vi "UHR-Fleezers Control (host) - 12.7.vi"() -> ()   [LabVIEW 2012] (continued)
              shift-left: _ -> [w2929]
              n2002 = case shown="True" w2938 {
                selector: w2938 -> [w2945 _]
                tunnel: w2940 -> [_ w2954]
                tunnel: w2939 -> [_ w2952]
                tunnel: [w2945 w2950] -> w2937
                tunnel: [w2944 w2949] -> w2936
                tunnel: [w2943 w2948] -> w2935
                tunnel: [w2942 w2947] -> w2934
                tunnel: [w2941 w2946] -> w2933
                tunnel: w2932 -> [w2944 _]
                tunnel: w2931 -> [w2943 _]
                tunnel: w2930 -> [w2942 _]
                tunnel: w2929 -> [w2941 _]
                frame False {
                }
                frame True {
                  n2003 = Unbundle(w2954) -> (w2953:T33)
                  n2004 = call "isclickinwindow.vi"("Image Param"=w2953, "Point32"=w2952) -> ("4 Y"=w2946:i32, "3 Height"=w2947:i32, "2 X"=w2948:i32, "1 Width"=w2949:i32, "In image?"=w2951:bool)  [unwired: 1 in]
                  n2005 = Not(x=w2951) -> (.not. x?=w2950:bool)
                }
              }
            }
            n2006 = Not(x=w2904) -> (.not. x?=w2903:bool)
            n2007 = case shown="True" w2903 {
              tunnel: w2901 -> [_ w2968]
              tunnel: w2899 -> [_ w2967]
              tunnel: w2902 -> [_ w2966]
              tunnel: w2900 -> [_ w2965]
              frame False {
              }
              frame True {
                w2955 = FALSE ("Get Point")
                n2008 = local read "Scan lines (y)"() -> (w2970:u64)
                n2009 = disable-structure shown="Disabled" {
                  frame Disabled {
                  }
                  frame Enabled {
                  }
                }
                n2010 = local read "Actual MCL Inc (V)"() -> (w2964:dbl)
                n2011 = local read "Scan steps (MCL)"() -> (w2969:u64)
                n2012 = Divide "Y Pix/step"(x=w2965, y=w2970) -> (x/y=w2977:dbl)
                n2013 = Divide "Y V/pix"(x=w2964, y=w2977) -> (x/y=w2976:dbl)
                n2014 = Divide "Y half step offset"(x=w2964, y=2.0) -> (x/y=w2978:dbl)
                n2015 = Divide "X pix/step"(x=w2966, y=w2969) -> (x/y=w2975:dbl)
                n2016 = Negate(x=w2978) -> (-x=w2979:dbl)
                n2017 = local read "Initial Y"() -> (w2985:dbl)
                n2018 = Multiply(x=w2967, y=w2976) -> (x*y=w2986:dbl)
                n2019 = Divide "X half step offset"(x=w2964, y=2.0) -> (x/y=w2972:dbl)
                n2020 = Divide "X V/pix"(x=w2964, y=w2975) -> (x/y=w2974:dbl)
                n2021 = Multiply(x=w2964, y=w2969) -> (x*y=w2981:dbl)
                n2022 = Compound Arithmetic op=ADD(w2979, w2986, w2985) -> (w2956:dbl)
                "Pointer Y (V)" <- w2956
                n2023 = Multiply(x=w2974, y=w2968) -> (x*y=w2983:dbl)
                n2024 = Negate(x=w2972) -> (-x=w2971:dbl)
                n2025 = local read "Initial X"() -> (w2984:dbl)
                n2026 = Negate(x=w2983) -> (-x=w2982:dbl)
                n2027 = Compound Arithmetic op=ADD(w2971, w2981, w2984, w2982) -> (w2957:dbl)
                "Pointer X (V)" <- w2957
                n2028 = case shown="True" "Set High F Confocal Spot (X-Y)" {
                  tunnel: w2957 -> [_ w2987]
                  tunnel: w2956 -> [_ w2988]
                  frame False {
                  }
                  frame True {
                    "Confocal Y 2 (V)" <- w2988
                    "Confocal X 2 (V)" <- w2987
                  }
                }
                n2029 = Or(x="Set X Only", y="Set Confocal Spot (X-Y)") -> (x .or. y?=w2960:bool)
                n2030 = Or(x="Set Confocal Spot (X-Y)", y="Set Y Only") -> (x .or. y?=w2959:bool)
                n2031 = case shown="True" w2960 {
                  tunnel: w2957 -> [_ w2989]
                  frame False {
                  }
                  frame True {
                    n2032 = property on="AO2" class="Slide (strict)"("Val(Sgnl)"=w2989) -> ()  [unwired: 2 in, 2 out]
                    "Confocal X 1 (V)" <- w2989
                  }
                }
                n2033 = case shown="True" w2959 {
                  tunnel: w2956 -> [_ w2990]
                  frame False {
                  }
                  frame True {
                    n2034 = property on="AO1" class="Slide (strict)"("Val(Sgnl)"=w2990) -> ()  [unwired: 2 in, 2 out]
                    "Confocal Y 1 (V)" <- w2990
                  }
                }
                n2035 = local write "Set High F Confocal Spot (X-Y)"(w2955) -> ()
                n2036 = local write "Set Confocal Spot (X-Y)"(w2955) -> ()
                n2037 = local write "Set X Only"(w2955) -> ()
                n2038 = local write "Set Y Only"(w2955) -> ()
              }
            }
          }
          frame 3 {
            n2039 = local read "BD 2 Frequency 1 (MHz)"() -> (w2991:dbl)
            n2040 = local read "BD 1 Frequency 1 (MHz)"() -> (w2992:dbl)
            n2041 = local write "Manipulating Trap"(TRUE ("Manipulating Trap")) -> ()
            n2042 = local write "Coords"(T7 {"Horizontal"=0, "Vertical"=0} ("Coords")) -> ()
            n2043 = while {
              tunnel: w2997 -> [w3002]
              tunnel: w2995 -> [w3001]
              tunnel: w2993 -> [w3000]
              tunnel: w2992 -> [w2999]
              tunnel: w2991 -> [w2998]
              stop <- w3003 stop-if-true
              n2044 = event shown="[0] \"Pane\": Mouse Move" {
                selector: _ -> [_ _]
                dyn-events: _ -> [_ _]
                timeout: _ -> [_ _]
                tunnel: ["Force Manip Abort" w3067] -> w3003
                tunnel: w3002 -> [w3010 _]
                tunnel: w3001 -> [w3008 _]
                tunnel: w3000 -> [w3007 _]
                tunnel: w2999 -> [w3006 _]
                tunnel: w2998 -> [w3005 _]
                event Mouse Move {
                  n2045 = event-data() -> ("Time"=w3011:u32, "Coords"=w3012:T7)  [unwired: 3 out]
                  n2046 = Less?(x=w3011, y=w3010) -> (x < y?=w3009:bool)
                  n2047 = case "Makes sure old motion events prior to mouse click aren't used" shown="False" w3009 {
                    tunnel: w3012 -> [w3054 _]
                    tunnel: w3008 -> [w3055 _]
                    tunnel: w3007 -> [w3032 _]
                    tunnel: w3006 -> [w3028 _]
                    tunnel: w3005 -> [w3027 _]
                    frame False {
                      n2048 = Subtract(x=w3054, y=w3055) -> (x-y=w3053:T7)
                      "Coords" <- w3053
                      n2049 = local read "Y RF Frequency Limits (MHz)"() -> (w3013:T16)
                      n2050 = To Double Precision Float(number=w3053) -> (double precision float=w3052:cluster{"Horizontal":dbl, "Vertical":dbl})
                      n2051 = Multiply(x=cluster{"Horizontal":dbl, "Vertical":dbl} {"Horizontal"=-1.0, "Vertical"=1.0}, y="Manipulation Scaling") -> (x*y=w3048:cluster{"Horizontal":dbl, "Vertical":dbl})
                      n2052 = local read "X RF Frequency Limits (MHz)"() -> (w3014:T16)
                      n2053 = Multiply(x=w3052, y=w3048) -> (x*y=w3050:cluster{"Horizontal":dbl, "Vertical":dbl})
                      n2054 = Unbundle By Name(w3050) -> ("Horizontal"=w3045:dbl, "Vertical"=w3049:dbl)
                      n2055 = Unbundle By Name(w3013) -> ("Maximum"=w3016:dbl, "Minimum"=w3015:dbl)
                      n2056 = Boolean To (0,1)(Boolean="Manip. X?") -> (0, 1=w3043:i16)
                      n2057 = Boolean To (0,1)(Boolean="Manip. Y?") -> (0, 1=w3040:i16)
                      n2058 = local read "BD 1 Frequency 2 (MHz)"() -> (w3030:dbl)
                      n2059 = Multiply(x=w3049, y=w3040) -> (x*y=w3042:dbl)
                      n2060 = Multiply(x=w3043, y=w3045) -> (x*y=w3046:dbl)
                      n2061 = local read "BD 2 Frequency 2 (MHz)"() -> (w3029:dbl)
                      n2062 = Unbundle By Name(w3014) -> ("Maximum"=w3018:dbl, "Minimum"=w3017:dbl)
                      n2063 = Add(x=w3027, y=w3042) -> (x+y=w3020:dbl)
                      n2064 = Add(x=w3028, y=w3046) -> (x+y=w3022:dbl)
                      n2065 = In Range and Coerce(upper limit=w3018, x=w3022, lower limit=w3017) -> (coerced(x)=w3021:dbl)  [unwired: 1 out]
                      n2066 = In Range and Coerce(upper limit=w3016, x=w3020, lower limit=w3015) -> (coerced(x)=w3019:dbl)  [unwired: 1 out]
                      n2067 = Subtract(x=w3021, y=w3030) -> (x-y=w3039:dbl)
                      n2068 = Subtract(x=w3019, y=w3029) -> (x-y=w3038:dbl)
                      n2069 = Square(x=w3039) -> (x^2=w3037:dbl)
                      n2070 = Square(x=w3038) -> (x^2=w3036:dbl)
                      n2071 = Add(x=w3037, y=w3036) -> (x+y=w3035:dbl)
                      n2072 = Square Root(x=w3035) -> (sqrt(x)=w3031:dbl)
                      n2073 = In Range and Coerce(upper limit="Limit Max (MHz)", x=w3031, lower limit="Limit Min (MHz)") -> (In Range?=w3024:bool)  [unwired: 1 out]
                      n2074 = Not(x="Limits Enable") -> (.not. x?=w3023:bool)
                      n2075 = Or(x=w3024, y=w3023) -> (x .or. y?=w3025:bool)
                      n2076 = case shown="True" w3025 {
                        tunnel: w3032 -> [_ w3065]
                        tunnel: w3031 -> [_ w3056]
                        tunnel: w3021 -> [_ w3063]
                        tunnel: w3030 -> [_ w3062]
                        tunnel: w3019 -> [_ w3061]
                        tunnel: w3029 -> [_ w3060]
                        tunnel: w3014 -> [_ w3058]
                        tunnel: w3013 -> [_ w3057]
                        frame False {
                        }
                        frame True {
                          n2077 = local read "BD 1 Frequency 3 (MHz)"() -> (w3064:dbl)
                          n2078 = local read "BD 2 Frequency 3 (MHz)"() -> (w3059:dbl)
                          n2079 = local write "Trap Delta (MHz)"(w3056) -> ()
                          n2080 = call "set RF board frequency - interlace.vi"("Board 2 Frequency Limits"=w3057, "Board 1 Frequency Limits"=w3058, "FPGA VI Reference In"=w3065, "Board 2 Frequency 3 (MHz)"=w3059, "Board 1 Frequency 3 (MHz)"=w3064, "Board 2 Frequency 2 (MHz)"=w3060, "Board 2 Frequency 1 (MHz)"=w3061, "Board 1 Frequency 2 (MHz)"=w3062, "Board 1 Frequency 1  (MHz)"=w3063) -> ()  [unwired: 1 in, 2 out]
                          n2081 = local write "BD 2 Frequency 1 (MHz)"(w3061) -> ()
                          n2082 = local write "BD 1 Frequency 1 (MHz)"(w3063) -> ()
                        }
                      }
                    }
                    frame True {
                    }
                  }
                }
                event Mouse Up {
                  n2083 = event-data() -> ("Button"=w3066:u16)  [unwired: 8 out]
                  n2084 = case shown="3" w3066 {
                    tunnel: [FALSE TRUE] -> w3067
                    frame 0, Default {
                    }
                    frame 3 {
                      n2085 = local read "Trap Delta (MHz)"() -> (w3069:dbl)
                      n2086 = property on="Initial delta (MHz)" class="DigNum (strict)"("Val(Sgnl)"=w3069) -> ()  [unwired: 2 in, 2 out]
                      n2087 = local write "Manipulating Trap"(FALSE ("Manipulating Trap")) -> ()
                    }
                  }
                }
              }
            }
          }
        }
      }
      event Mouse Move {
        n2088 = event-data() -> ()  [unwired: 6 out]
      }
    }
    n2089 = local read "Stop All"() -> (w2885:bool)
    n2090 = node-c288() -> ()  [unwired: 2 out]
  }
  n2091 = timed-loop "Main data acquisition loop (get data, process data for display, and save data to disk)" {
    tunnel: w17 -> [w3381]
    tunnel: w89 -> [w3380]
    tunnel: [w3410] -> w293
    tunnel: [w3405] -> w291
    timing: w201 -> [_]
    timing-out: [_] -> w200
    tunnel: w106 -> [w3234]
    stop <- "Stop All" stop-if-true
    w3151 = "Initialize"
    # "Fluorescence data into FIFO for external control vi's\n(e.g., fluorescence triggering) - Duncan Nall"
    n2092 = node-c288() -> ()  [unwired: 2 out]
    n2093 = First Call?() -> (First Call?: T/F=w3186:bool)
    n2094 = Or(x="Reset", y=w3186) -> (x .or. y?=w3187:bool)
    n2095 = local read "Flushing P1"() -> (w3106:bool)
    n2096 = case "Reset data stream (manual reset or at begining of some rastering and imaging)" shown="True" w3187 {
      tunnel: w3381 -> [w4451 w4459]
      tunnel: w3380 -> [w4450 w4458]
      tunnel: [w4451 w4453] -> w3376
      tunnel: [w4450 w4452] -> w3375
      frame False {
      }
      frame True {
        w4456 = TRUE ("AI to FIFO")
        n2097 = local write "Overflow (data lost)"(FALSE ("Overflow (data lost)")) -> ()
        n2098 = call "reset FPGA DMA.vi"("error in"=w4458, "FPGA VI Reference In"=w4459) -> ("error out"=w4454:errorcluster, "FPGA VI Reference Out"=w4455:T20)
        n2099 = xnode "Read/Write Control"("FPGA VI Reference In"=w4455, "error in"=w4454, "AI to FIFO"=w4456, "APD to FIFO"=w4456) -> ("FPGA VI Reference Out"=w4453:T20, "error out"=w4452:errorcluster)
      }
    }
    n2100 = case shown="True" w3106 {
      frame False {
      }
      frame True {
        n2101 = local read "Flush rate (uL/m) P1"() -> (w3440:dbl)
        n2102 = local read "HP1 Flush Time (s)"() -> (w3449:dbl)
        n2103 = local read "DMA Update Period (s)"() -> (w3443:dbl)
        n2104 = Divide(x=w3440, y=60.0) -> (x/y=w3441:dbl)
        n2105 = Divide(x=w3449, y=w3443) -> (x/y=w3438:dbl)
        n2106 = feedback #1(0) -> (w3447:i32)
        n2107 = Increment(x=w3447) -> (x+1=w3437:i32)
        n2108 = Greater?(x=w3437, y=w3438) -> (0:w3446:bool)
        n2109 = Compound Arithmetic op=MULTIPLY(w3443, w3437, w3441) -> (→"P1 Flush Volume (uL)":dbl)
        n2110 = Divide(x=w3437, y=w3438) -> (x/y=→"P1 Flushing Bar":dbl)
        n2111 = case shown="True" w3446 {
          tunnel: w3437 -> [w3450 _]
          tunnel: [w3450 0] -> w3445
          frame False {
          }
          frame True {
            w3451 = FALSE ("Flushing P1")
            n2112 = local write "Inject Pump 1"(w3451) -> ()
            n2113 = local write "Flushing P1"(w3451) -> ()
            n2114 = property on="Clear Volume P1" class="Bool (strict)"("Val(Sgnl)"=TRUE ("Value (Signaling)")) -> ()  [unwired: 2 in, 2 out]
          }
        }
        n2115 = feedback-in #1(w3445) -> ()
      }
    }
    n2116 = Or(x="Start AOD Scan", y="Trap Raster Scan") -> (x .or. y?=w3332:bool)
    n2117 = case "Start AOM raster scan" shown="True" w3332 {
      tunnel: w3376 -> [w4301 w4311]
      tunnel: w3375 -> [w4300 w4310]
      tunnel: [w4301 w4304] -> w3374
      tunnel: [w4300 w4303] -> w3373
      frame False {
      }
      frame True {
        n2118 = case shown="True" "Restart DMA? (AOD)" {
          tunnel: [w4349 w4351] -> w4305
          tunnel: [w4348 w4350] -> w4306
          tunnel: w4311 -> [w4349 w4353]
          tunnel: w4310 -> [w4348 w4352]
          frame False {
          }
          frame True {
            n2119 = local write "Overflow (data lost)"(FALSE ("Overflow (data lost)")) -> ()
            n2120 = call "reset FPGA DMA.vi"("error in"=w4352, "FPGA VI Reference In"=w4353) -> ("error out"=w4350:errorcluster, "FPGA VI Reference Out"=w4351:T20)
          }
        }
        n2121 = local write "Trap Raster Scan"(FALSE ("Trap Raster Scan")) -> ()
        n2122 = case shown="True" "Move MCL Also?" {
          tunnel: w4306 -> [w4314 w4343]
          tunnel: w4305 -> [w4315 w4344]
          tunnel: [w4313 w4347] -> w4304
          tunnel: [w4312 w4346] -> w4303
          frame False {
            w4316 = TRUE ("AI to FIFO")
            n2123 = xnode "Read/Write Control"("FPGA VI Reference In"=w4315, "error in"=w4314, "AI to FIFO"=w4316, "APD to FIFO"=w4316, "Start scan"=w4316) -> ("FPGA VI Reference Out"=w4313:T20, "error out"=w4312:errorcluster)
          }
          frame True {
            w4340 = FALSE ("1D or 2D Scan?")
            w4345 = TRUE ("AI to FIFO")
            # "Count for MCL loop"
            # "N total cycles"
            # "N steps"
            # "V_int"
            n2124 = local read "Scan Range (nm)"() -> (w4322:dbl)
            n2125 = local read "Number of F/B Scans (AOD)"() -> (w4339:u16)
            n2126 = Sign(1:w4322) -> (0:w4321:dbl)
            n2127 = Compound Arithmetic op=MULTIPLY(w4322, "MCL Step Position Ratio", "MCL/AOM Scale Tweak") -> (w4326:dbl)
            n2128 = Negate(x=w4321) -> (-x=w4318:dbl)
            n2129 = Multiply(x=w4318, y="MCL Step Increment (V_int)") -> (x*y=w4320:dbl)
            n2130 = Divide(x=w4326, y="MCL X Cal (nm/V)") -> (x/y=w4332:dbl)
            n2131 = Multiply(x=32767.0 ("y"), y=w4332) -> (x*y=w4338:dbl)
            n2132 = local read "Total Counts (ticks)"() -> (w4323:u16)
            n2133 = local read "Cycles/step (AOD)"() -> (w4334:u64)
            n2134 = local read "Scan steps (AOD)"() -> (w4335:u64)
            n2135 = Divide(x=w4338, y=10.0) -> (x/y=w4331:dbl)
            n2136 = Divide(x=w4331, y="MCL Step Increment (V_int)") -> (x/y=w4329:dbl)
            n2137 = Absolute Value(x=w4329) -> (abs(x)=w4317:dbl)
            n2138 = Compound Arithmetic op=MULTIPLY(w4335, w4334, w4323) -> (w4330:u64)
            n2139 = local write "wait to reset values"(w4345) -> ()
            n2140 = local write "MCL Scanning"(w4345) -> ()
            n2141 = Divide(x=w4330, y=w4317) -> (x/y=w4327:dbl)
            "MCL Count" <- w4327
            n2142 = xnode "Read/Write Control"("FPGA VI Reference In"=w4344, "error in"=w4343, "Scan steps (MCL)"=w4317, "Number of scans (MCL)"=w4339, "Cycles per step (MCL)"=u64 1, "Scan freq.  increment (MCL)"=w4320, "1D or 2D Scan?"=w4340, "MCL Scan Axis"=w4340, "Cont. Scan (MCL)"=w4340, "MCL count"=w4327) -> ("FPGA VI Reference Out"=w4342:T20, "error out"=w4341:errorcluster)
            n2143 = xnode "Read/Write Control"("FPGA VI Reference In"=w4342, "error in"=w4341, "AI to FIFO"=w4345, "APD to FIFO"=w4345, "Start scan"=w4345, "Start scan (MCL)"=w4345) -> ("FPGA VI Reference Out"=w4347:T20, "error out"=w4346:errorcluster)
          }
        }
        "Raster Scanning..." <- TRUE ("Scanning...")
      }
    }
    n2144 = local read "Flushing P3"() -> (w3107:bool)
    n2145 = case "Keep track of when Harvard Pump 3 is done flushing" shown="True" w3107 {
      frame False {
      }
      frame True {
        n2146 = local read "Flush rate (uL/m) P3"() -> (w3457:dbl)
        n2147 = local read "DMA Update Period (s)"() -> (w3459:dbl)
        n2148 = local read "HP3 Flush Time (s)"() -> (w3466:dbl)
        n2149 = Divide(x=w3457, y=60.0) -> (x/y=w3455:dbl)
        n2150 = feedback #2(0) -> (w3464:i32)
        n2151 = Increment(x=w3464) -> (x+1=w3458:i32)
        n2152 = Divide(x=w3466, y=w3459) -> (x/y=w3460:dbl)
        n2153 = Greater?(x=w3458, y=w3460) -> (0:w3463:bool)
        n2154 = Compound Arithmetic op=MULTIPLY(w3459, w3458, w3455) -> (→"P3 Flush Volume (uL)":dbl)
        n2155 = case shown="True" w3463 {
          tunnel: w3458 -> [w3467 _]
          tunnel: [w3467 0] -> w3462
          frame False {
          }
          frame True {
            w3468 = FALSE ("Flushing P3")
            n2156 = local write "Inject Pump 3"(w3468) -> ()
            n2157 = local write "Flushing P3"(w3468) -> ()
            n2158 = property on="Clear Volume P3" class="Bool (strict)"("Val(Sgnl)"=TRUE ("Value (Signaling)")) -> ()  [unwired: 2 in, 2 out]
          }
        }
        n2159 = feedback-in #2(w3462) -> ()
        n2160 = Divide(x=w3458, y=w3460) -> (x/y=→"P3 Flushing Bar":dbl)
      }
    }
    n2161 = And(x="Save scans", y=w3332) -> (x .and. y?=w3372:bool)
    n2162 = Compound Arithmetic op=OR("Start MCL Scan", "Confocal Image", "Confocal Linescan") -> (w3330:bool)
    n2163 = And(x="Save Data (MCL)", y=w3330) -> (x .and. y?=w3371:bool)
    n2164 = case "Start MCL raster scan" shown="True" w3330 {
      tunnel: w3374 -> [w3913 w3929]
      tunnel: w3373 -> [w3912 w3928]
      tunnel: [w3913 w3924] -> w3233
      tunnel: [w3912 w3923] -> w3232
      tunnel: [FALSE w3922] -> w3357
      tunnel: "Start MCL Scan" -> [_ w3917]
      tunnel: "Confocal Image" -> [_ w3916]
      tunnel: "Confocal Linescan" -> [_ _]
      frame False {
      }
      frame True {
        w3922 = TRUE
        n2165 = case shown="True" "Restart DMA? (MCL)" {
          tunnel: [w3974 w3976] -> w3927
          tunnel: [w3973 w3975] -> w3926
          tunnel: w3929 -> [w3974 w3979]
          tunnel: w3928 -> [w3973 w3978]
          frame False {
          }
          frame True {
            n2166 = call "reset FPGA DMA.vi"("error in"=w3978, "FPGA VI Reference In"=w3979) -> ("error out"=w3975:errorcluster, "FPGA VI Reference Out"=w3976:T20)
            n2167 = local write "Overflow (data lost)"(FALSE ("Overflow (data lost)")) -> ()
          }
        }
        n2168 = case shown="False" w3917 {
          selector: w3917 -> [_ w3933]
          tunnel: w3916 -> [w3932 _]
          tunnel: [w3932 w3933] -> w3915
          frame False {
            n2169 = property on="2D or 1D Scan" class="Bool (strict)"("Val(Sgnl)"=w3932) -> ()  [unwired: 2 in, 2 out]
            n2170 = property on="Confocal Image" class="Bool (strict)"("Value"=FALSE ("Start Confocal Map")) -> ()  [unwired: 2 in, 2 out]
          }
          frame True {
          }
        }
        n2171 = local write "MCL Scanning"(w3922) -> ()
        n2172 = local read "AO1"() -> (w3919:dbl)
        n2173 = local read "AO2"() -> (w3918:dbl)
        n2174 = case shown="True" "Center Scan" {
          tunnel: w3927 -> [w3940 w3972]
          tunnel: w3926 -> [w3939 w3971]
          tunnel: [w3938 w3970] -> w3924
          tunnel: [w3937 w3969] -> w3923
          tunnel: [w3935 w3956] -> w3921
          tunnel: [w3934 w3955] -> w3920
          tunnel: w3919 -> [w3935 w3961]
          tunnel: w3918 -> [w3934 w3964]
          tunnel: w3915 -> [_ _]
          frame False {
            w3936 = TRUE ("AI to FIFO")
            n2175 = xnode "Read/Write Control"("FPGA VI Reference In"=w3940, "error in"=w3939, "AI to FIFO"=w3936, "APD to FIFO"=w3936, "Start scan (MCL)"=w3936) -> ("FPGA VI Reference Out"=w3938:T20, "error out"=w3937:errorcluster)
          }
          frame True {
            w3968 = TRUE ("AI to FIFO")
            n2176 = local read "Scan steps (MCL)"() -> (w3947:u64)
            n2177 = local read "Scan lines (y)"() -> (w3943:u64)
            n2178 = local read "Fast Scan Dir"() -> (w3954:bool)
            n2179 = local read "Actual MCL Inc (V)"() -> (w3944:dbl)
            n2180 = Decrement(x=w3943) -> (x-1=w3942:u64)
            n2181 = Decrement(x=w3947) -> (x-1=w3946:u64)
            n2182 = Multiply(x=w3944, y=w3942) -> (x*y=w3941:dbl)
            n2183 = Divide(x=w3941, y=2.0) -> (x/y=w3951:dbl)
            n2184 = Multiply(x=w3944, y=w3946) -> (x*y=w3945:dbl)
            n2185 = Divide(x=w3945, y=2.0) -> (x/y=w3950:dbl)
            n2186 = Select(t=w3950, s=w3954, f=w3951) -> (s? t:f=w3949:dbl)
            n2187 = Select(t=w3951, s=w3954, f=w3950) -> (s? t:f=w3953:dbl)
            n2188 = Subtract(x=w3961, y=w3953) -> (x-y=w3952:dbl)
            n2189 = Subtract(x=w3964, y=w3949) -> (x-y=w3948:dbl)
            n2190 = local read "2D or 1D Scan"() -> (w3966:bool)
            n2191 = Not(x=w3954) -> (.not. x?=w3960:bool)
            n2192 = Not(x=w3966) -> (.not. x?=w3962:bool)
            n2193 = And(x=w3954, y=w3962) -> (x .and. y?=w3963:bool)
            n2194 = And(x=w3962, y=w3960) -> (x .and. y?=w3965:bool)
            n2195 = Select(t=w3964, s=w3965, f=w3948) -> (s? t:f=w3955:dbl)
            n2196 = Select(t=w3961, s=w3963, f=w3952) -> (s? t:f=w3956:dbl)
            n2197 = call "Volt to I16.vi"("Voltage In"=w3956) -> ("I16 Voltage Out"=w3959:i16)
            n2198 = call "Volt to I16.vi"("Voltage In"=w3955) -> ("I16 Voltage Out"=w3958:i16)
            n2199 = xnode "Read/Write Control"("FPGA VI Reference In"=w3972, "error in"=w3971, "AI to FIFO"=w3968, "APD to FIFO"=w3968, "Start scan (MCL)"=w3968, "AO1"=w3959, "AO2"=w3958) -> ("FPGA VI Reference Out"=w3970:T20, "error out"=w3969:errorcluster)
          }
        }
        "Initial Y" <- w3921
        "Initial X" <- w3920
        n2200 = local write "Tab Control 6"(T3."Imaging" ("Tab Control 6")) -> ()
        "wait to reset values" <- w3922
      }
    }
    n2201 = local read "APD Elements/DMA read"() -> (w3074:u32)
    n2202 = local read "Trap AI Elements/DMA read"() -> (w3295:u32)
    n2203 = xnode "Get APD Data"("FPGA VI Reference In"=w3233, "error in"=w3232, "Number of Elements"=w3074, "Timeout (ms)"=-1) -> ("Data"=w3264:u32[], "Elements Remaining"=→"APD FIFO Elements Remaining":u32)  [unwired: 2 out]
    n2204 = local read "Trap Pos Elements/DMA read"() -> (w3229:u32)
    n2205 = xnode "Invoke Method"("FPGA VI Reference In"=w3233, "error in"=w3232, "Number of Elements"=w3229, "Timeout (ms)"=-1) -> ("Data"=w3193:u16[], "Elements Remaining"=→"Trap Pos FIFO El Remaining":u32)  [unwired: 2 out]
    n2206 = xnode "Get Trap Data"("FPGA VI Reference In"=w3233, "error in"=w3232, "Number of Elements"=w3295, "Timeout (ms)"=-1 ("Timeout")) -> ("FPGA VI Reference Out"=w3128:T20, "error out"=w3127:errorcluster, "Data"=w3194:i16[], "Elements Remaining"=w3418:u32)
    "FIFO El. Rem." <- w3418
    n2207 = local read "DMA Update Period (s)"() -> (w3296:dbl)
    n2208 = local read "Trap AI FIFO Depth"() -> (w3420:u32)
    n2209 = local read "Number of APDs"() -> (w3096:u8)
    n2210 = Decimate 1D Array(w3193) -> (w3190:u16[], w3192:u16[], w3191:u16[])
    n2211 = feedback #3(0.0) -> (w3222:dbl)
    n2212 = Add(x=w3296, y=w3222) -> (x+y=w3394:dbl)
    n2213 = feedback-in #3(w3394) -> ()
    n2214 = To Time Stamp(1:w3222) -> (0:w3221:timestamp)
    n2215 = Subtract(x=w3420, y=w3295) -> (x-y=w3419:u32)
    n2216 = To Unsigned Long Integer(number=w3190) -> (unsigned 32bit integer=w3189:u32[])
    n2217 = Join Numbers(hi=w3192, lo=w3191) -> ((hi.lo)=w3188:u32[])
    n2218 = Divide(x=w3418, y=w3419) -> (x/y=w3417:dbl)
    "Buffer Status" <- w3417
    n2219 = case "Deinterlace APD signals" shown="3, Default" w3096 {
      tunnel: [w3430 w3436] -> w3073
      tunnel: w3264 -> [w3431 w3435]
      tunnel: [w3429 w3434] -> w3072
      tunnel: [w3428 w3432] -> w3079
      frame 3, Default {
        n2220 = Decimate 1D Array "APD signals"(w3431) -> (w3430:u32[], w3429:u32[], w3428:u32[])
      }
      frame 2 {
        n2221 = Decimate 1D Array "APD signals"(w3435) -> (w3436:u32[], w3434:u32[])
        n2222 = Multiply(x=w3434, y=u32 0) -> (x*y=w3432:u32[])
      }
    }
    n2223 = Join Numbers(hi=w3189, lo=w3188) -> ((hi.lo)=w3182:u64[])
    n2224 = call "IR AOM word to freq - vec.vi"("Frequency Word In (double vec)"=w3182) -> ("Frequency Out"=w3228:dbl[])
    n2225 = Equal?(x=w3417, y=1.0) -> (x = y?=w3415:bool)
    n2226 = case "Alert buffer overflow" shown="True" w3415 {
      frame False {
      }
      frame True {
        n2227 = call <vilib>:"Beep.vi"() -> ()  [unwired: 3 in, 9 out]
        "Overflow (data lost)" <- TRUE ("Overflow (data lost)")
      }
    }
    n2228 = Decimate 1D Array(w3228) -> (w3227:dbl[], w3226:dbl[])
    n2229 = Build Array(w3227, w3226) -> (w3225:dbl[][])
    n2230 = Bundle(w3073, w3072, w3079) -> (w3077:cluster{u32[], u32[], u32[]})  [unwired: 1 in]
    n2231 = Build Array(w3073, w3072, w3079) -> (w3354:u32[][])
    n2232 = for {
      tunnel: w3073 -> [w3426] mode=indexing
      n2233 = call "Smart Buffer (DBL) 1.vi"("new element [write]"=w3426, "mode"=T21."write") -> ()  [unwired: 4 in, 6 out]
    }
    n2234 = local read "APD Integration Time (s)"() -> (w3089:dbl)
    n2235 = To Double Precision Float(number=w3354) -> (double precision float=w3355:dbl[][])
    n2236 = feedback #4 "APD3"(w3079) -> (w3095:u32[])
    n2237 = feedback #5 "APD2"(w3072) -> (w3251:u32[])
    n2238 = feedback #6 "APD1"(w3073) -> (w3353:u32[])
    n2239 = Build Array (concatenate)(w3251, w3072) -> (w3250:u32[])
    n2240 = Build Array (concatenate)(w3095, w3079) -> (w3094:u32[])
    n2241 = Build Array (concatenate)(w3353, w3073) -> (w3350:u32[])
    n2242 = for {
      tunnel: w3072 -> [w3425] mode=indexing
      n2243 = call "Smart Buffer (DBL) 2.vi"("new element [write]"=w3425, "mode"=T21."write") -> ()  [unwired: 4 in, 6 out]
    }
    n2244 = Array Size(array=w3350) -> (size(s)=w3347:i32)
    n2245 = Array Size(array=w3073) -> (size(s)=w3349:i32)
    n2246 = Multiply(x=w3349, y="APD Ave N") -> (x*y=w3348:dbl)
    n2247 = Greater?(x=w3347, y=w3348) -> (0:w3351:bool)
    n2248 = Bundle("APD 1", "APD 2", "APD 3") -> (w3387:cluster{string, string, string})  [unwired: 1 out]
    n2249 = local read "Trap Sets"() -> (w3294:u32)
    n2250 = case shown="True" w3351 {
      tunnel: w3350 -> [w3728 w3737]
      tunnel: [w3728 w3735] -> w3301
      tunnel: w3348 -> [_ w3730]
      tunnel: w3347 -> [_ w3736]
      tunnel: w3250 -> [w3727 w3734]
      tunnel: [w3727 w3733] -> w3248
      tunnel: w3094 -> [w3726 w3732]
      tunnel: [w3726 w3729] -> w3090
      frame False {
      }
      frame True {
        n2251 = Subtract(x=w3736, y=w3730) -> (x-y=w3731:dbl)
        n2252 = Array Subset "APD3"(array=w3732, index=w3731, length=w3730) -> (w3729:u32[])
        n2253 = Array Subset "APD2"(array=w3734, index=w3731, length=w3730) -> (w3733:u32[])
        n2254 = Array Subset "APD1"(array=w3737, index=w3731, length=w3730) -> (w3735:u32[])
      }
    }
    n2255 = feedback-in #4(w3090) -> ()
    n2256 = feedback-in #5(w3248) -> ()
    n2257 = feedback-in #6(w3301) -> ()
    n2258 = Cluster To Array(cluster=w3387) -> (array=w3384:string[])
    n2259 = for "APD" {
      tunnel: w3355 -> [w3984] mode=indexing
      tunnel: w3089 -> [w3991]
      tunnel: [w3987] -> w3252 mode=indexing
      tunnel: "APD Disp. Scale" -> [w3988]
      tunnel: w3384 -> [w3986] mode=indexing
      tunnel: "APD Disp. Downsample" -> [w3982]
      tunnel: [w3985] -> w3383
      workers-P: _ -> [_]
      tunnel: w3221 -> [w3981]
      n2260 = call "integrate 1D array interval - double.vi"("Ave N"=w3982, "Array In"=w3984) -> ("Array Out"=w3983:dbl[])  [unwired: 1 out]
      n2261 = Multiply(x=w3991, y=w3982) -> (x*y=w3985:dbl)
      n2262 = Divide(x=w3983, y=w3988) -> (x/y=w3989:dbl[])
      n2263 = Bundle By Name("t0"=w3981, "Y"=w3989, "dt"=w3985) -> (w3990:waveform(dbl))  [unwired: 1 out]
      n2264 = Set Waveform Attribute(5:w3986, 6:"NI_ChannelName" ("name"), 7:w3990) -> (3:w3987:waveform(dbl))  [unwired: 1 in, 2 out]
    }
    "APD Display Period (s)" <- w3383
    n2265 = Reciprocal(x=w3383) -> (1/x=→"APD Display Freq. (Hz)":dbl)
    n2266 = case "Deinterlace trap data, average down PSD" shown="2" w3294 {
      tunnel: w3194 -> [w4009 w4074]
      tunnel: [w4006 w4071] -> w3287
      tunnel: [w4009 w4073] -> w3185
      tunnel: "Detector Type" -> [w4008 w4069]
      tunnel: [w4007 w4072] -> w3286
      tunnel: [w4005 w4070] -> w3392
      frame 1, Default {
        n2267 = Divide(x=w4009, y=3276.7) -> (x/y=w4010:dbl[])
        n2268 = Decimate 1D Array(w4010) -> (w4019:dbl[], w4018:dbl[], w4017:dbl[], w4016:dbl[], w4015:dbl[], w4014:dbl[], w4013:dbl[], w4012:dbl[])
        n2269 = case shown="\"IR-QPD + PSD + FB-QPD position\"" w4008 {
          tunnel: w4019 -> [w4043 w4068]
          tunnel: w4018 -> [w4042 w4067]
          tunnel: w4017 -> [w4027 w4045]
          tunnel: w4016 -> [w4028 w4055]
          tunnel: w4015 -> [w4041 w4066]
          tunnel: w4014 -> [w4040 w4065]
          tunnel: w4013 -> [w4024 w4046]
          tunnel: w4012 -> [w4023 w4044]
          tunnel: [w4022 w4052] -> w4007
          tunnel: [w4021 w4051] -> w4006
          tunnel: [w4020 w4050] -> w4005
          frame "IR-QPD + PSD + FB-QPD", Default {
            w4020 = 0  # Channel pattern
            n2270 = Divide(x=w4043, y=w4028) -> (x/y=w4030:dbl[])
            n2271 = Divide(x=w4042, y=w4028) -> (x/y=w4029:dbl[])
            n2272 = Divide(x=w4041, y=w4024) -> (x/y=w4026:dbl[])
            n2273 = Divide(x=w4040, y=w4023) -> (x/y=w4025:dbl[])
            n2274 = Build Array(w4030, w4029, w4028, w4027, w4026, w4025, w4024, w4023) -> (w4021:dbl[][])
            n2275 = Bundle("T1 Y", "T1 X", "T1 Sum", "FB Sum", "PSD Y", "PSD X", "PSD Y Sum", "PSD X Sum") -> (w4039:T41)  [unwired: 1 out]
            n2276 = Cluster To Array(cluster=w4039) -> (array=w4022:string[])
          }
          frame "IR-QPD + PSD + FB-QPD position" {
            w4050 = 3  # Channel pattern
            n2277 = Negate(x=w4046) -> (-x=w4047:dbl[])
            n2278 = Divide(x=w4068, y=w4055) -> (x/y=w4057:dbl[])
            n2279 = Divide(x=w4067, y=w4055) -> (x/y=w4056:dbl[])
            n2280 = Divide(x=w4066, y=w4046) -> (x/y=w4054:dbl[])
            n2281 = Divide(x=w4065, y=w4047) -> (x/y=w4053:dbl[])
            n2282 = Build Array(w4057, w4056, w4055, w4044, w4045, w4054, w4053, w4046) -> (w4051:dbl[][])
            n2283 = Bundle("T1 Y", "T1 X", "T1 Sum", "FB X", "FB Sum", "PSD Y", "PSD X", "PSD Y Sum") -> (w4064:T41)  [unwired: 1 out]
            n2284 = Cluster To Array(cluster=w4064) -> (array=w4052:string[])
          }
        }
      }
      frame 2 {
        n2285 = case shown="\"IR-QPD + PSD + FB-QPD X position\"" w4069 {
          tunnel: w4074 -> [w4136 w4208 w4279]
          tunnel: [w4075 w4199 w4210] -> w4073
          tunnel: [w4102 w4190 w4257] -> w4072
          tunnel: [w4101 w4153 w4224] -> w4071
          tunnel: [w4095 w4188 w4255] -> w4070
          frame "IR-QPD + PSD + FB-QPD", Default {
            w4095 = 1  # Channel pattern
            # "time average x2 the 4th signal and the 4 psd signals (detection laser)"
            # "deinterlace 3 signals from qpd"
            n2286 = Decimate 1D Array(w4136) -> (w4135:i16[], w4134:i16[], w4100:i16[], w4133:i16[], w4123:i16[], w4121:i16[], w4120:i16[], w4118:i16[])
            n2287 = Decimate 1D Array(w4100) -> (w4099:i16[], w4098:i16[])
            n2288 = Decimate 1D Array(w4135) -> (w4132:i16[], w4104:i16[])
            n2289 = Decimate 1D Array(w4134) -> (w4131:i16[], w4129:i16[])
            n2290 = Decimate 1D Array(w4133) -> (w4130:i16[], w4128:i16[])
            n2291 = call "downsample 1D array - double.vi"("Ave N"=2.0, "Array In"=w4123) -> ("Array Out"=w4122:dbl[])  [unwired: 1 out]
            n2292 = call "downsample 1D array - double.vi"("Ave N"=2.0, "Array In"=w4121) -> ("Array Out"=w4103:dbl[])  [unwired: 1 out]
            n2293 = call "downsample 1D array - double.vi"("Ave N"=2.0, "Array In"=w4120) -> ("Array Out"=w4119:dbl[])  [unwired: 1 out]
            n2294 = call "downsample 1D array - double.vi"("Ave N"=2.0, "Array In"=w4118) -> ("Array Out"=w4117:dbl[])  [unwired: 1 out]
            n2295 = Interleave 1D Arrays(w4132, w4131, w4130, w4104, w4129, w4128, w4099, w4098, w4122, w4103, w4119, w4117) -> (w4116:dbl[])
            n2296 = Divide(x=w4116, y=3276.7) -> (x/y=w4115:dbl[])
            n2297 = Decimate 1D Array(w4115) -> (w4114:dbl[], w4113:dbl[], w4112:dbl[], w4111:dbl[], w4110:dbl[], w4109:dbl[], w4097:dbl[], w4096:dbl[], w4108:dbl[], w4107:dbl[], w4106:dbl[], w4105:dbl[])
            n2298 = Divide(x=w4114, y=w4112) -> (x/y=w4082:dbl[])
            n2299 = Divide(x=w4113, y=w4112) -> (x/y=w4081:dbl[])
            n2300 = Divide(x=w4111, y=w4109) -> (x/y=w4080:dbl[])
            n2301 = Divide(x=w4110, y=w4109) -> (x/y=w4079:dbl[])
            n2302 = Divide(x=w4108, y=w4106) -> (x/y=w4078:dbl[])
            n2303 = Divide(x=w4107, y=w4105) -> (x/y=w4077:dbl[])
            n2304 = Build Array(w4082, w4081, w4112, w4080, w4079, w4109, w4097, w4096, w4078, w4077, w4106, w4105) -> (w4101:dbl[][])
            n2305 = Bundle("T1 Y", "T1 X", "T1 Sum", "T2 Y", "T2 X", "T2 Sum", "T1 FB Sum", "T2 FB Sum", "PSD Y", "PSD X", "PSD Y Sum", "PSD X Sum") -> (w4083:T42)  [unwired: 1 out]
            n2306 = To Word Integer(number=w4116) -> (16bit integer=w4075:i16[])
            n2307 = Cluster To Array(cluster=w4083) -> (array=w4102:string[])
          }
          frame "IR-QPD + PSD + FB-QPD X position" {
            w4188 = 2  # Channel pattern
            # "time average x2 the 3 psd signals (detection laser)"
            # "deinterlace 3 signals from qpds"
            n2308 = Decimate 1D Array(w4208) -> (w4207:i16[], w4206:i16[], w4189:i16[], w4205:i16[], w4151:i16[], w4148:i16[], w4145:i16[], w4176:i16[])
            n2309 = Select(t=i16 -1, s="Flip X Sign", f=i16 1) -> (s? t:f=w4141:i16)
            n2310 = Multiply(x=w4206, y=w4141) -> (x*y=w4142:i16[])
            n2311 = Decimate 1D Array(w4189) -> (w4174:i16[], w4172:i16[])
            n2312 = Decimate 1D Array(w4207) -> (w4204:i16[], w4191:i16[])
            n2313 = Decimate 1D Array(w4142) -> (w4203:i16[], w4201:i16[])
            n2314 = Decimate 1D Array(w4205) -> (w4202:i16[], w4200:i16[])
            n2315 = Decimate 1D Array(w4176) -> (w4175:i16[], w4173:i16[])
            n2316 = call "downsample 1D array - I16.vi"("Ave N"=2.0, "Array In"=w4151) -> ("Array Out"=w4149:i16[])  [unwired: 1 in]
            n2317 = call "downsample 1D array - I16.vi"("Ave N"=2.0, "Array In"=w4145) -> ("Array Out"=w4143:i16[])  [unwired: 1 in]
            n2318 = call "downsample 1D array - I16.vi"("Ave N"=2.0, "Array In"=w4148) -> ("Array Out"=w4146:i16[])  [unwired: 1 in]
            n2319 = Interleave 1D Arrays(w4204, w4203, w4202, w4191, w4201, w4200, w4175, w4174, w4173, w4172, w4149, w4146, w4143) -> (w4199:i16[])
            n2320 = Divide(x=w4199, y=3276.7) -> (x/y=w4198:dbl[])
            n2321 = Decimate 1D Array(w4198) -> (w4197:dbl[], w4196:dbl[], w4195:dbl[], w4194:dbl[], w4193:dbl[], w4192:dbl[], w4164:dbl[], w4162:dbl[], w4161:dbl[], w4159:dbl[], w4158:dbl[], w4157:dbl[], w4154:dbl[])
            n2322 = Negate(x=w4154) -> (-x=w4152:dbl[])
            n2323 = Divide(x=w4158, y=w4154) -> (x/y=w4156:dbl[])
            n2324 = Divide(x=w4157, y=w4152) -> (x/y=w4155:dbl[])
            n2325 = Divide(x=w4197, y=w4195) -> (x/y=w4180:dbl[])
            n2326 = Divide(x=w4196, y=w4195) -> (x/y=w4179:dbl[])
            n2327 = Divide(x=w4194, y=w4192) -> (x/y=w4178:dbl[])
            n2328 = Divide(x=w4193, y=w4192) -> (x/y=w4177:dbl[])
            n2329 = Divide(x=w4164, y=w4162) -> (x/y=w4163:dbl[])
            n2330 = Divide(x=w4161, y=w4159) -> (x/y=w4160:dbl[])
            n2331 = Build Array(w4180, w4179, w4195, w4178, w4177, w4192, w4163, w4162, w4160, w4159, w4156, w4155, w4154) -> (w4153:dbl[][])
            n2332 = Bundle("T1 Y", "T1 X", "T1 Sum", "T2 Y", "T2 X", "T2 Sum", "T1 FB X", "T1 FB Sum", "T2 FB X", "T2 FB Sum", "PSD Y", "PSD X", "PSD Y Sum") -> (w4181:T43)  [unwired: 1 out]
            n2333 = Cluster To Array(cluster=w4181) -> (array=w4190:string[])
          }
          frame "IR-QPD + PSD + FB-QPD XY positions" {
            w4255 = 4  # Channel pattern
            # "time average x2 the 3 psd signals (detection laser)"
            # "deinterlace 3 signals from qpds"
            n2334 = Decimate 1D Array(w4279) -> (w4278:i16[], w4277:i16[], w4256:i16[], w4276:i16[], w4222:i16[], w4268:i16[], w4267:i16[], w4244:i16[])
            n2335 = Decimate 1D Array "Feedback Sum"(w4256) -> (w4240:i16[], w4238:i16[])
            n2336 = Decimate 1D Array "QPD Y"(w4278) -> (w4275:i16[], w4258:i16[])
            n2337 = Decimate 1D Array "QPD X"(w4277) -> (w4274:i16[], w4272:i16[])
            n2338 = Decimate 1D Array "Feedback Y"(w4222) -> (w4221:i16[], w4220:i16[])
            n2339 = Decimate 1D Array "QPD Sum"(w4276) -> (w4273:i16[], w4271:i16[])
            n2340 = Decimate 1D Array "Feedback X"(w4244) -> (w4241:i16[], w4239:i16[])
            n2341 = call "downsample 1D array - double.vi"("Ave N"=2.0, "Array In"=w4268) -> ("Array Out"=w4243:dbl[])  [unwired: 1 out]
            n2342 = call "downsample 1D array - double.vi"("Ave N"=2.0, "Array In"=w4267) -> ("Array Out"=w4242:dbl[])  [unwired: 1 out]
            n2343 = Interleave 1D Arrays(w4275, w4274, w4273, w4258, w4272, w4271, w4221, w4241, w4240, w4220, w4239, w4238, w4243, w4242) -> (w4266:dbl[])
            n2344 = Divide(x=w4266, y=3276.7) -> (x/y=w4265:dbl[])
            n2345 = Decimate 1D Array(w4265) -> (w4264:dbl[], w4263:dbl[], w4262:dbl[], w4261:dbl[], w4260:dbl[], w4259:dbl[], w4217:dbl[], w4231:dbl[], w4215:dbl[], w4216:dbl[], w4229:dbl[], w4213:dbl[], w4227:dbl[], w4225:dbl[])
            n2346 = Negate(x=w4225) -> (-x=w4223:dbl[])
            n2347 = Divide(x=w4227, y=w4223) -> (x/y=w4226:dbl[])
            n2348 = Divide(x=w4216, y=w4213) -> (x/y=w4212:dbl[])
            n2349 = Divide(x=w4217, y=w4215) -> (x/y=w4214:dbl[])
            n2350 = Divide(x=w4264, y=w4262) -> (x/y=w4248:dbl[])
            n2351 = Divide(x=w4263, y=w4262) -> (x/y=w4247:dbl[])
            n2352 = Divide(x=w4261, y=w4259) -> (x/y=w4246:dbl[])
            n2353 = Divide(x=w4260, y=w4259) -> (x/y=w4245:dbl[])
            n2354 = Divide(x=w4231, y=w4215) -> (x/y=w4230:dbl[])
            n2355 = Divide(x=w4229, y=w4213) -> (x/y=w4228:dbl[])
            n2356 = Build Array(w4248, w4247, w4262, w4246, w4245, w4259, w4214, w4230, w4215, w4212, w4228, w4213, w4226, w4225) -> (w4224:dbl[][])
            n2357 = Bundle("T1 Y", "T1 X", "T1 Sum", "T2 Y", "T2 X", "T2 Sum", "T1 FB Y", "T1 FB X", "T1 FB Sum", "T2 FB Y", "T2 FB X", "T2 FB Sum", "PSD X", "PSD Y Sum") -> (w4211:T44)  [unwired: 1 out]
            n2358 = To Word Integer(number=w4266) -> (16bit integer=w4210:i16[])
            n2359 = Cluster To Array(cluster=w4211) -> (array=w4257:string[])
          }
        }
      }
    }
    "AI labels" <- w3286
    n2360 = local read "APD Integration Time (s)"() -> (w3259:dbl)
    n2361 = Array Size(array=w3301) -> (size(s)=w3346:i32)
    n2362 = call <vilib>:"Std Deviation and Variance.vi"("X"=w3248) -> ("standard deviation"=w3247:dbl)  [unwired: 1 in, 2 out]
    n2363 = Add Array Elements(numeric array=w3248) -> (sum=w3249:u32)
    n2364 = Add Array Elements(numeric array=w3301) -> (sum=w3356:u32)
    n2365 = call <vilib>:"Std Deviation and Variance.vi"("X"=w3301) -> ("standard deviation"=w3300:dbl)  [unwired: 1 in, 2 out]
    n2366 = Divide(x=w3247, y=w3089) -> (x/y=w3244:dbl)
    "Rate sigma (Hz) 2" <- w3244
    n2367 = Multiply(x=w3089, y=w3346) -> (x*y=w3091:dbl)
    "Int. Time (s)" <- w3091
    n2368 = Divide(x=w3249, y=w3091) -> (x/y=w3245:dbl)
    "APD 2 Rate (Hz)" <- w3245
    n2369 = Multiply(x="APD Disp. Scale", y=w3252) -> (x*y=w3261:waveform(dbl)[])
    n2370 = Divide(x=w3356, y=w3091) -> (x/y=w3298:dbl)
    "APD 1 Rate (Hz)" <- w3298
    n2371 = Divide(x=w3300, y=w3089) -> (x/y=w3299:dbl)
    "Rate sigma (Hz)" <- w3299
    n2372 = Divide(x=w3244, y=w3245) -> (x/y=→"Sigma/Mean 2":dbl)
    n2373 = Multiply(x="APD Disp. Downsample", y=w3259) -> (x*y=w3257:dbl)
    n2374 = Divide(x=w3299, y=w3298) -> (x/y=→"Sigma/Mean":dbl)
    n2375 = Divide(x=w3261, y=w3257) -> (x/y=w3081:waveform(dbl)[])
    n2376 = Index Array(array=w3081, index=0) -> (element=w3241:waveform(dbl))
    n2377 = Index Array(array=w3081, index=1) -> (element=w3239:waveform(dbl))
    n2378 = Index Array(array=w3081, index=2) -> (element=w3083:waveform(dbl))
    n2379 = Subtract(x=w3241, y="APD 1 Offset") -> (x-y=w3237:waveform(dbl))
    n2380 = Subtract(x=w3239, y="APD 2 Offset") -> (x-y=w3236:waveform(dbl))
    n2381 = Subtract(x=w3083, y="APD 3 Offset") -> (x-y=w3080:waveform(dbl))
    n2382 = Add Array Elements(numeric array=w3090) -> (sum=w3093:u32)
    n2383 = call <vilib>:"Std Deviation and Variance.vi"("X"=w3090) -> ("standard deviation"=w3092:dbl)  [unwired: 1 in, 2 out]
    n2384 = Build Array(w3237, w3236, w3080) -> (→"APD Chart":waveform(dbl)[])
    n2385 = Divide(x=w3093, y=w3091) -> (x/y=w3087:dbl)
    "APD 3 Rate (Hz)" <- w3087
    n2386 = Divide(x=w3092, y=w3089) -> (x/y=w3088:dbl)
    "Rate sigma (Hz) 3" <- w3088
    n2387 = Divide(x=w3088, y=w3087) -> (x/y=→"Sigma/Mean 3":dbl)
    n2388 = local read "Data Period (s)"() -> (w3144:dbl)
    n2389 = local read "BD 1 Frequency 2 (MHz)"() -> (w3177:dbl)
    n2390 = local read "BD 1 Frequency 1 (MHz)"() -> (w3178:dbl)
    n2391 = Decimate 1D Array(w3185) -> (w3209:i16[], w3208:i16[], w3206:i16[], w3205:i16[])  [unwired: 9 out]
    n2392 = Multiply(x=w3144, y="Trap Pos. Disp. Downsample") -> (x*y=w3142:dbl)
    n2393 = Divide(x=w3209, y=w3208) -> (x/y=w3210:dbl[])
    n2394 = Divide(x=w3206, y=w3205) -> (x/y=w3207:dbl[])
    n2395 = local read "AOM X Cal (nm/MHz)"() -> (w3175:dbl)
    n2396 = Split 1D Array(array=w3210, index="N El. to Ave.") -> (second subarray=w3213:dbl[])  [unwired: 1 out]
    n2397 = Split 1D Array(array=w3207, index="N El. to Ave.") -> (second subarray=w3212:dbl[])  [unwired: 1 out]
    n2398 = Multiply(x=w3144, y="Trap Disp. Downsample") -> (x*y=w3223:dbl)
    "Display Period (s)" <- w3223
    n2399 = for "Trap AI" {
      tunnel: [w4004] -> w3388 mode=indexing
      tunnel: w3221 -> [w3995]
      tunnel: "Trap Disp. Downsample" -> [w4002]
      tunnel: w3287 -> [w4000] mode=indexing
      tunnel: w3144 -> [w3999]
      tunnel: w3286 -> [w3998] mode=indexing
      tunnel: [w3997] -> w3256 mode=indexing
      tunnel: w3223 -> [w3996]
      workers-P: _ -> [_]
      n2400 = Bundle By Name("Y"=w4000, "dt"=w3999) -> (w4001:waveform(dbl))  [unwired: 1 out]
      n2401 = Set Waveform Attribute(5:w3998, 6:"NI_ChannelName" ("name"), 7:w4001) -> (3:w3997:waveform(dbl))  [unwired: 1 in, 2 out]
      n2402 = call "downsample 1D array - double.vi"("Ave N"=w4002, "Array In"=w4000) -> ("Array Out"=w4003:dbl[])  [unwired: 1 out]
      n2403 = Bundle By Name(cluster=w3997, "t0"=w3995, "Y"=w4003, "dt"=w3996) -> (w4004:waveform(dbl))
    }
    n2404 = Bundle("BD 1 Frequency 1 (MHz)"=w3178, "BD 1 Frequency 2 (MHz)"=w3177) -> (w3179:T45)  [unwired: 1 out]
    n2405 = call-poly <vilib>:"Mean.vi"("X"=w3212) -> ("mean"=w3200:dbl)  [unwired: 1 out]
    n2406 = call-poly <vilib>:"Mean.vi"("X"=w3213) -> ("mean"=w3201:dbl)  [unwired: 1 out]
    n2407 = Reciprocal(x=w3223) -> (1/x=→"Trap Disp. Freq. (Hz)":dbl)
    n2408 = Cluster To Array(cluster=w3179) -> (array=w3176:dbl[])
    n2409 = local read "Trap X AI1 (DMA)"() -> (w3211:T13)
    n2410 = local read "Data points/scans (MCL)"() -> (w3366:dbl)
    n2411 = To Fixed-Point(number=w3200) -> (fixed-point=w3198:fxp<+/-,16,1>)  [unwired: 1 in]
    n2412 = To Fixed-Point(number=w3201) -> (fixed-point=w3199:fxp<+/-,16,1>)  [unwired: 1 in]
    n2413 = Bundle("Trap 1 Pos.", "Trap 2 Pos.") -> (w3220:cluster{string, string})  [unwired: 1 out]
    n2414 = Bundle By Name(cluster=w3211, "Set 1"=w3199, "Set 2"=w3198) -> (→"Trap X AI1 (DMA)":T13)
    n2415 = Cluster To Array(cluster=w3220) -> (array=w3217:string[])
    n2416 = Unbundle(w3077) -> (w3078:u32[])  [unwired: 2 out]
    n2417 = Select(t=-1.0, s="Negate Y Axis", f=1.0) -> (s? t:f=w3161:dbl)
    n2418 = for "Trap Position" {
      tunnel: w3225 -> [w3596] mode=indexing
      tunnel: "Trap Pos. Disp. Downsample" -> [w3595]
      tunnel: w3142 -> [w3593]
      tunnel: w3221 -> [w3592]
      tunnel: w3217 -> [w3590] mode=indexing
      tunnel: [w3589] -> w3131 mode=indexing
      tunnel: w3176 -> [w3587] mode=indexing
      tunnel: w3175 -> [w3585]
      tunnel: w3161 -> [w3584]
      n2419 = call "downsample 1D array - double.vi"("Ave N"=w3595, "Array In"=w3596) -> ("Array Out"=w3594:dbl[])  [unwired: 1 out]
      n2420 = Subtract(x=w3594, y=w3587) -> (x-y=w3588:dbl[])
      n2421 = Multiply(x=w3585, y=w3588) -> (x*y=w3586:dbl[])
      n2422 = Multiply(x=w3584, y=w3586) -> (x*y=w3583:dbl[])
      n2423 = Bundle By Name("Y"=w3583, "dt"=w3593, "t0"=w3592) -> (w3591:waveform(dbl))  [unwired: 1 out]
      n2424 = Set Waveform Attribute(5:w3590, 6:"NI_ChannelName" ("name"), 7:w3591) -> (3:w3589:waveform(dbl))  [unwired: 1 in, 2 out]
    }
    n2425 = To Double Precision Float(number=w3078) -> (double precision float=w3284:dbl[])
    n2426 = local read "Display Period (s)"() -> (w3273:dbl)
    n2427 = Increment(x=w3366) -> (x+1=w3367:dbl)
    n2428 = Index Array(array=w3131, index=0) -> (element=w3135:waveform(dbl))
    n2429 = Index Array(array=w3131, index=1) -> (element=w3130:waveform(dbl))
    n2430 = feedback #7(w3367) -> (w3370:dbl)
    n2431 = Select(t=0, s=w3357, f=w3370) -> (s? t:f=w3363:dbl)
    n2432 = Array Size(array=w3284) -> (size(s)=w3369:i32)
    n2433 = Build Array (concatenate)(w3252, w3388) -> (w3254:waveform(dbl)[])
    "All Signals" <- w3254
    n2434 = Add(x=w3369, y=w3363) -> (x+y=w3364:dbl)
    n2435 = Unbundle By Name(w3135) -> ("Y"=w3136:dbl[])
    n2436 = Divide(x="Bead Sep. Int. Time (s)", y=w3273) -> (x/y=w3171:dbl)
    n2437 = Add(x=w3136, y="FB Trap Pos Offset") -> (x+y=w3134:dbl[])
    "T1 x pos data" <- w3134
    n2438 = Greater?(x=w3364, y=w3366) -> (0:w3365:bool)
    n2439 = feedback #8(w3134) -> (w3173:dbl[])
    n2440 = Build Array (concatenate)(w3134, w3173) -> (w3172:dbl[])
    n2441 = Bundle By Name(cluster=w3135, "Y"=w3134) -> (w3133:waveform(dbl))
    n2442 = Select(t=w3363, s=w3365, f=w3364) -> (s? t:f=w3362:dbl)
    n2443 = feedback-in #7(w3362) -> ()
    n2444 = local read "MCL Scanning"() -> (w3360:bool)
    n2445 = Bundle(w3133, w3130) -> (w3129:cluster{waveform(dbl), waveform(dbl)})  [unwired: 1 out]
    n2446 = Split 1D Array(array=w3172, index=w3171) -> (first subarray=w3165:dbl[])  [unwired: 1 out]
    n2447 = feedback-in #8(w3165) -> ()
    n2448 = Not(x=w3365) -> (.not. x?=w3359:bool)
    n2449 = Cluster To Array(cluster=w3129) -> (array=w3105:waveform(dbl)[])
    "Trap Positions" <- w3105
    n2450 = call-poly <vilib>:"Mean.vi"("X"=w3165) -> ("mean"=w3164:dbl)  [unwired: 1 out]
    "Mean T1 Position (nm)" <- w3164
    n2451 = Subtract(x=w3165, y=w3164) -> (x-y=w3170:dbl[])
    n2452 = Square(x=w3170) -> (x^2=w3169:dbl[])
    n2453 = And(x=w3359, y=w3360) -> (x .and. y?=w3361:bool)
    n2454 = call-poly <vilib>:"Mean.vi"("X"=w3169) -> ("mean"=w3168:dbl)  [unwired: 1 out]
    n2455 = Square Root(x=w3168) -> (sqrt(x)=w3167:dbl)
    n2456 = Or(x=w3361, y=w3357) -> (x .or. y?=w3358:bool)
    n2457 = Equal?(x="Tab Control 6", y=T35."High Res Display") -> (x = y?=w3290:bool)
    n2458 = Multiply(x=10.0, y=w3167) -> (x*y=→"Trap 1 Position RMS (A)":dbl)
    n2459 = case "For displaying the high resolution display (no downsampling)" shown="True" w3290 {
      tunnel: w3256 -> [_ w3616]
      frame False {
      }
      frame True {
        n2460 = Index Array(array=w3616, index="High Res. Display") -> (element=w3617:waveform(dbl))
        n2461 = call <vilib>:"Std Deviation and Variance.vi"("X"=w3617) -> ("mean"=w3624:dbl, "standard deviation"=w3629:dbl)  [unwired: 1 in, 1 out]
        "Mean Intensity" <- w3624
        "Sigma" <- w3629
        n2462 = Subtract(x=w3617, y=w3624) -> (x-y=w3623:waveform(dbl))
        n2463 = Select(t=w3623, s="Subtract mean", f=w3617) -> (s? t:f=→"1 Channel":waveform(dbl))
        n2464 = Divide(x=w3629, y=w3624) -> (x/y=→"Sigma/Mean":dbl)
        n2465 = feedback #9(1) -> (w3618:i32)
        n2466 = Greater Or Equal?(x=w3618, y="Slow mean N ave.") -> (x >= y?=w3631:bool)
        n2467 = Increment(x=w3618) -> (x+1=w3633:i32)
        n2468 = Select(t=1, s=w3631, f=w3633) -> (s? t:f=w3620:i32)
        n2469 = feedback-in #9(w3620) -> ()
        n2470 = feedback #10() -> (w3621:waveform(dbl))  [unwired: 1 out]
        n2471 = case shown="Default" w3618 {
          tunnel: [w3636 w3639] -> w3622
          tunnel: w3621 -> [w3638 _]
          tunnel: w3617 -> [w3637 w3639]
          frame Default {
            n2472 = call-poly <vilib>:"Append Waveforms.vi"("waveform B"=w3637, "waveform A"=w3638) -> ("waveform out"=w3636:waveform(dbl))  [unwired: 1 in, 8 out]
          }
          frame 1 {
          }
        }
        n2473 = feedback-in #10(w3622) -> ()
        n2474 = case shown="True" w3631 {
          tunnel: w3622 -> [_ w3635]
          frame False {
          }
          frame True {
            n2475 = call-poly <vilib>:"Mean.vi"("X"=w3635) -> ("mean"=→"Slow mean":dbl)  [unwired: 1 out]
          }
        }
      }
    }
    n2476 = case "For plotting results of scanning MCL (fluorescence and detection laser images)" shown="True" w3358 {
      tunnel: w3357 -> [_ w3743]
      tunnel: w3366 -> [_ _]
      tunnel: w3256 -> [_ w3872]
      tunnel: w3234 -> [_ w3780]
      tunnel: w3077 -> [_ w3750]
      frame False {
      }
      frame True {
        w3760 = u32 0 items=["Horizontal", "Vertical", "Central", "1st Diagonal", "2nd Diagonal"] ("Type of Symmetry")
        w3787 = u32 0 items=["Horizontal", "Vertical", "Central", "1st Diagonal", "2nd Diagonal"] ("Type of Symmetry")
        w3811 = u32 0 items=["Horizontal", "Vertical", "Central", "1st Diagonal", "2nd Diagonal"] ("Type of Symmetry")
        w3814 = u32 0 items=["Horizontal", "Vertical", "Central", "1st Diagonal", "2nd Diagonal"] ("Type of Symmetry")
        w3843 = u32 0 items=["Horizontal", "Vertical", "Central", "1st Diagonal", "2nd Diagonal"] ("Type of Symmetry")
        n2477 = Unbundle(w3750) -> (w3749:u32[], w3747:u32[], w3745:u32[])
        n2478 = To Double Precision Float(number=w3749) -> (double precision float=w3748:dbl[])